vi "ImageAnalysis.vi"(9 "Background Image":dbl[][](graph)=array1004x1002[1006008 elements], 10 "Atom Image":dbl[][](graph)=array1004x1002[1006008 elements]) -> ()   [LabVIEW 2013]
uses:
  Controls/ExperimentParameters/experimentalvariables.ctl
panel:
  in  "Experimental Variables":T1={"Electronic Background to Subtract from\nimages"=500.0, "Pixel Size before binning (µm)"=14.2, "Imaging Wavelength (m)"=4.61e-07, "Isotope"=84, "1P1 Linewidth (MHz)"=32.0} {"Isotope" min=84 max=88; "Imaging Wavelength (m)" format="%#_6p"}
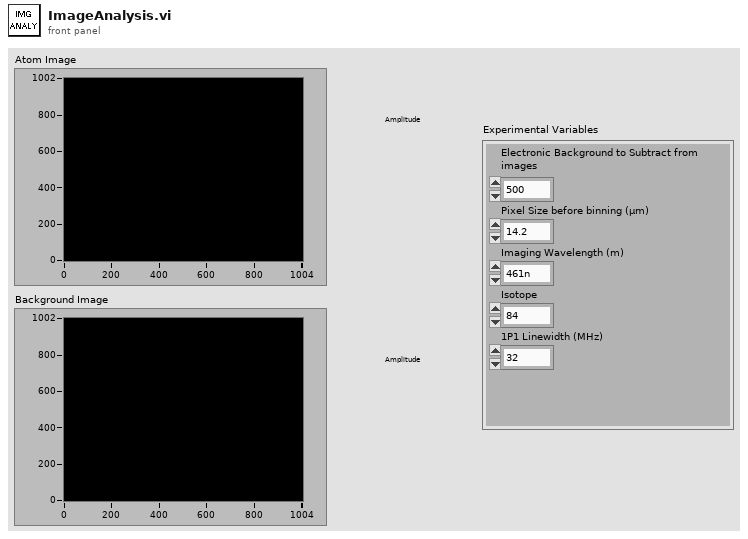
[diagram p1: front panel]
types:
  T1 = typedef "experimentalvariables.ctl" = cluster{"Electronic Background to Subtract from\nimages":dbl, "Pixel Size before binning (µm)":dbl, "Imaging Wavelength (m)":dbl, "Isotope":i32, "1P1 Linewidth (MHz)":dbl}
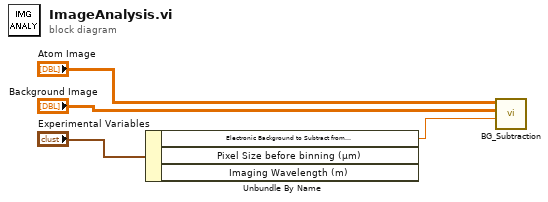
[diagram p0: block diagram]
diagram:
  n1 = Unbundle By Name("Experimental Variables") -> ("Electronic Background to Subtract from\nimages"=w1:dbl)  [unwired: 2 out]
  n2 = call "BG_Subtraction.vi"("Electronic Background to Subtract"=w1, "Background Image"="Background Image", "Atom Image"="Atom Image") -> ()  [unwired: 6 in, 3 out]
